vi "HFRR ADV v041.vi"() -> ()   [LabVIEW 2025] (continued)
            n1752 = property on="Port 3" class="Bool (strict)"("Visible"=w2089) -> ()  [unwired: 2 in, 2 out]
          }
        }
        n1753 = Wait (ms)(milliseconds to wait=u32 40) -> ()  [unwired: 1 out]
        n1754 = case shown="True" w2074 {
          tunnel: [w2086 errorcluster {"status"=TRUE, "code"=0, "source"="Init"} ("error out")] -> w2075
          tunnel: w2078 -> [w2086 _]
          frame False {
          }
          frame True {
          }
        }
        n1755 = case shown="Error" w2075 {
          selector: w2075 -> [w2096 w2114]
          tunnel: [w2099 w2118] -> w2085
          tunnel: [w2098 w2112] -> w2084
          tunnel: w2076 -> [w2097 w2116]
          frame No Error {
            n1756 = property class="Instr"(reference=w2097, error in=w2096) -> (reference out=w2094:refnum<visa-resource-name>, error out=w2095:errorcluster, "Serial Settings:Number of Bytes at Serial Port"=w2091:u32)
            n1757 = Greater?(x=w2091, y=u32 5) -> (0:w2090:bool)
            n1758 = Not(x=w2090) -> (.not. x?=→"Port 1a":bool)
            n1759 = while {
              tunnel: [w2107] -> w2098
              tunnel: [w2106] -> w2099
              tunnel: w2095 -> [w2105]
              tunnel: w2094 -> [w2104]
              stop <- TRUE stop-if-true
              n1760 = property class="Instr" props=["Serial Settings:Number of Bytes at Serial Port"](reference=w2104, error in=w2105) -> (reference out=w2109:refnum<visa-resource-name>, error out=w2108:errorcluster)  [unwired: 1 out]
              n1761 = VISA Read(VISA resource name=w2109, byte count=u32 50, error in (no error)=w2108) -> (VISA resource name out=w2106:refnum<visa-resource-name>, read buffer=w2101:string, error out=w2107:errorcluster)  [unwired: 1 out]
              n1762 = Wait (ms)(milliseconds to wait=u32 5) -> ()  [unwired: 1 out]
            }
          }
          frame Error {
            w2124 = u16 0 items=["None", "XON/XOFF", "RTS/CTS", "XON/XOFF & RTS/CTS", "DTR/DSR", "XON/XOFF & DTR/DSR"] ("flow control (0:none)  2")
            w2122 = u16 10 items=["1.0"=10, "1.5"=15, "2.0"=20] ("stop bits 2")
            w2120 = u16 0 items=["None", "Odd", "Even", "Mark", "Space"] ("parity 2")
            w2121 = u32 10000  # timeout (10sec)
            n1763 = VISA Close(VISA resource name=w2116, error in (no error)=w2114) -> (error out=w2117:errorcluster)
            n1764 = local write "Port 1a"(FALSE ("Port 1a")) -> ()
            n1765 = local read "Com Port 1"() -> (w2111:refnum<visa-resource-name>)
            n1766 = call <vilib>:"Clear Errors.vi"("error in (no error)"=w2117) -> ("error out"=w2115:errorcluster)  [unwired: 5 in, 1 out]
            n1767 = call-poly "VISA Configure Serial Port"("VISA resource name"=w2111, "timeout (10sec)"=w2121, "baud rate (9600)"=u32 250000 ("baud rate  2"), "data bits (8)"=u16 8 ("data bits  2"), "parity (0:none)"=w2120, "error in (no error)"=w2115, "stop bits (10: 1 bit)"=w2122, "flow control (0:none)"=w2124) -> ("VISA resource name out"=w2125:refnum<visa-resource-name>, "error out"=w2126:errorcluster)  [unwired: 6 in]
            n1768 = flat-sequence {
              tunnel: w2125 -> [w2128]
              tunnel: w2126 -> [w2127]
              tunnel: [w2128] -> w2118
              tunnel: [w2127] -> w2112
              frame #0 {
                n1769 = Wait (ms)(milliseconds to wait=u32 50) -> ()  [unwired: 1 out]
              }
            }
            "Residual Uno" <- ""
          }
        }
        n1770 = local read "Quit"() -> (w2073:bool)
        "Error Uno" <- w2078
      }
      n1771 = VISA Close(VISA resource name=w2071, error in (no error)=w2070) -> (error out=w2068:errorcluster)
      n1772 = call <vilib>:"Clear Errors.vi"("error in (no error)"=w2068) -> ()  [unwired: 5 in, 2 out]
    }
    frame Enabled {
    }
  }
  n1773 = while {
    stop <- w2139 stop-if-true
    # "V0OLTAGE TO STROKE (peice vise calibration)"
    n1774 = local read "LVDT MIN"() -> (w2131:dbl)
    n1775 = local read "LVDT Peak"() -> (w2130:dbl)
    n1776 = Wait (ms)(milliseconds to wait=u32 10) -> ()  [unwired: 1 out]
    n1777 = formula code="// Dynamic Parameterized Linear Interpolation Node\n// Inputs: vpp_val, voltages (Array), distances (Array)\n// Outputs: stroke\n\nint i = 0;\nint segments = 11; // 12 points make 11 interpolation segments\n\n// 1. Lower Boundary Clamp\nif (vpp_val <= voltages[0]) {\n    stroke = distances[0];\n}\n// 2. Upper Boundary Clamp\nelse if (vpp_val >= voltages[segments]) {\n    stroke = distances[segments];\n}\n// 3. Dynamic Segment Search Loop\nelse {\n    stroke = distances[0]; // Fallback baseline\n    for (i = 0; i < segments; i++) {\n        if (vpp_val >= voltages[i] && vpp_val <= voltages[i+1]) {\n            // Standard linear interpolation formula using array lookups\n            stroke = distances[i] + (vpp_val - voltages[i]) * (distances[i+1] - distances[i]) / (voltages[i+1] - voltages[i]);\n            break; // Segment found, safely exit the loop\n        }\n    }\n}"("vpp_val"=w2130, "voltages"="calibration values", "distances"="STROKE") -> ("stroke"=→"LVDT STROKE":dbl)
    n1778 = local read "Calibration Tare Value"() -> (w2135:dbl)
    n1779 = local read "Calibration Tare"() -> (w2133:bool)
    n1780 = Subtract(x=w2131, y=w2135) -> (x-y=→"LVDT STROKE  Calibration":dbl)
    n1781 = case shown="True" w2133 {
      selector: w2133 -> [_ w2141]
      tunnel: w2131 -> [_ w2142]
      frame False {
      }
      frame True {
        n1782 = Not(x=w2141) -> (.not. x?=w2140:bool)
        n1783 = local write "Calibration Tare"(w2140) -> ()
        "Calibration Tare Value" <- w2142
      }
    }
    n1784 = local read "Quit"() -> (w2139:bool)
  }
  n1785 = while {
    stop <- w2165 stop-if-true
    n1786 = local read "Due read"() -> (w2163:string)
    n1787 = call <vilib>:"High Resolution Polling Wait.vi"("seconds to wait"=0.02) -> ()  [unwired: 10 in, 1 out]
    n1788 = local read "Frictioin Force Raw"() -> (w2145:dbl)
    n1789 = Spreadsheet String To Array(delimiter (Tab)=";", format string="", spreadsheet string=w2163, array type (2D Dbl)=string[] []) -> (array=w2160:string[])
    n1790 = Fract/Exp String To Number(string=w2160) -> (number=w2159:dbl[])  [unwired: 3 in, 1 out]
    n1791 = call <vilib>:"Median Filter PtByPt.vi"("rank"=2, "x"=w2145) -> ("Filtered x"=→"Friction":dbl)  [unwired: 2 in, 1 out]
    n1792 = Index Array(array=w2159) -> (element #1=→"Sample Temperature":dbl, element #2=→"Target Sample Temperature":dbl, element #3=→"Current Duty Cycle":dbl, element #4=→"Ambient Temperature":dbl, element #5=→"Dac Status":dbl, element #6=→"Vpp":dbl, element #7=→"Active Error Code":dbl, element #8=→"Kp":dbl, element #9=→"Ki":dbl, element #10=→"Kd":dbl, element #11=→"SampleRaw":dbl, element #12=→"AmbRaw":dbl)  [unwired: 12 in]
    n1793 = local read "Quit"() -> (w2165:bool)
  }
  n1794 = while {
    shift-right: [w2179] -> w43
    shift-left: _ -> [w2171]
    shift-right: [w2166] -> w42
    shift-left: errorcluster {"status"=FALSE, "code"=0, "source"="Init"} ("error out") -> [w2173]
    tunnel: [w2168] -> w46
    tunnel: [w2178] -> _
    i -> [w2178]
    stop <- w2168 stop-if-true
    n1795 = local read "Com Port 2"() -> (w2172:refnum<visa-resource-name>)
    n1796 = local read "Port 2a"() -> (w2174:bool)
    n1797 = Unbundle(w2173) -> ("status"=→"Port 4":bool)  [unwired: 2 out]
    n1798 = call <vilib>:"High Resolution Polling Wait.vi"("seconds to wait"=0.02) -> ()  [unwired: 10 in, 1 out]
    n1799 = local read "Port 4"() -> (w2175:bool)
    n1800 = Not Equal?(x=w2172, y=w2171) -> (x != y?=w2170:bool)
    n1801 = Or(x=w2175, y=w2174) -> (x .or. y?=w2177:bool)
    n1802 = case shown="False" w2177 {
      frame False {
        w2182 = TRUE ("Visible")
        n1803 = property on="Port 2a" class="Bool (strict)"("Visible"=w2182) -> ()  [unwired: 2 in, 2 out]
        n1804 = property on="Port 4" class="Bool (strict)"("Visible"=w2182) -> ()  [unwired: 2 in, 2 out]
      }
      frame True {
        w2183 = TRUE ("Visible")
        n1805 = property on="Port 2a" class="Bool (strict)"("Visible"=w2183) -> ()  [unwired: 2 in, 2 out]
        n1806 = property on="Port 4" class="Bool (strict)"("Visible"=w2183) -> ()  [unwired: 2 in, 2 out]
      }
    }
    n1807 = case shown="True" w2170 {
      tunnel: [w2180 errorcluster {"status"=TRUE, "code"=0, "source"="Init"} ("error out")] -> w2169
      tunnel: w2173 -> [w2180 _]
      frame False {
      }
      frame True {
      }
    }
    n1808 = case shown="No Error" w2169 {
      selector: w2169 -> [w2196 w2227]
      tunnel: [w2189 w2232] -> w2179
      tunnel: [w2197 w2225] -> w2166
      tunnel: w2171 -> [w2198 w2230]
      frame No Error {
        n1809 = property class="Instr" props=["Serial Settings:Number of Bytes at Serial Port"](reference=w2198, error in=w2196) -> (reference out=w2190:refnum<visa-resource-name>, error out=w2195:errorcluster)  [unwired: 1 out]
        n1810 = while {
          tunnel: [w2206] -> w2191
          tunnel: [w2205] -> w2192
          tunnel: w2195 -> [w2204]
          tunnel: w2190 -> [w2203]
          tunnel: [w2202] -> _
          i -> [w2202]
          stop <- TRUE stop-if-true
          n1811 = property class="Instr" props=["Serial Settings:Number of Bytes at Serial Port"](reference=w2203, error in=w2204) -> (reference out=w2208:refnum<visa-resource-name>, error out=w2207:errorcluster)  [unwired: 1 out]
          n1812 = VISA Read(VISA resource name=w2208, byte count=u32 1000, error in (no error)=w2207) -> (VISA resource name out=w2205:refnum<visa-resource-name>, read buffer=→"Due read":string, error out=w2206:errorcluster)  [unwired: 1 out]
        }
        n1813 = local read "Due Write"() -> (w2188:string)
        n1814 = call <vilib>:"Trim Whitespace.vi"("string"=w2188) -> ("trimmed string"=w2187:string)  [unwired: 1 in]
        n1815 = Not Equal?(x=w2187, y="") -> (x != y?=w2193:bool)
        n1816 = VISA Flush I/O Buffer(VISA resource name=w2192) -> (VISA resource name out=w2185:refnum<visa-resource-name>, error out=→"error out 10":errorcluster)  [unwired: 2 in]
        n1817 = case shown="True" w2193 {
          tunnel: w2185 -> [w2210 w2215]
          tunnel: [w2210 w2219] -> w2189
          tunnel: w2191 -> [w2209 w2214]
          tunnel: [w2209 w2217] -> w2197
          tunnel: w2187 -> [_ w2213]
          tunnel: [_ w2216] -> _
          frame False {
            # "DATA  WRITE LOOP"
          }
          frame True {
            n1818 = Concatenate Strings(w2213, "\r\n") -> (w2212:string)
            n1819 = VISA Write(VISA resource name=w2215, write buffer=w2212, error in (no error)=w2214) -> (VISA resource name out=w2219:refnum<visa-resource-name>, return count=w2216:u32, error out=w2218:errorcluster)
            n1820 = flat-sequence {
              tunnel: w2218 -> [w2221]
              tunnel: [w2221] -> w2217
              frame #0 {
                n1821 = local write "Due Write"("" ("Command")) -> ()
                n1822 = Wait (ms)(milliseconds to wait=u32 5) -> ()  [unwired: 1 out]
              }
            }
          }
        }
        "Port 2a" <- TRUE ("Port 2a")
      }
      frame Error {
        w2238 = u16 0 items=["None", "XON/XOFF", "RTS/CTS", "XON/XOFF & RTS/CTS", "DTR/DSR", "XON/XOFF & DTR/DSR"] ("flow control (0:none)  2")
        w2236 = u16 10 items=["1.0"=10, "1.5"=15, "2.0"=20] ("stop bits 2")
        w2234 = u16 0 items=["None", "Odd", "Even", "Mark", "Space"] ("parity 2")
        w2235 = u32 10000  # timeout (10sec)
        n1823 = VISA Clear(VISA resource name=w2230, error in (no error)=w2227) -> (VISA resource name out=w2229:refnum<visa-resource-name>, error out=w2228:errorcluster)
        n1824 = VISA Close(VISA resource name=w2229, error in (no error)=w2228) -> (error out=w2231:errorcluster)
        n1825 = call <vilib>:"Clear Errors.vi"("error in (no error)"=w2231) -> ()  [unwired: 5 in, 2 out]
        n1826 = local write "Port 2a"(FALSE ("Port 2a")) -> ()
        n1827 = local read "Com Port 2"() -> (w2224:refnum<visa-resource-name>)
        "visa due" <- w2224
        n1828 = call-poly "VISA Configure Serial Port"("VISA resource name"=w2224, "timeout (10sec)"=w2235, "baud rate (9600)"=u32 250000 ("baud rate  2"), "data bits (8)"=u16 8 ("data bits  2"), "parity (0:none)"=w2234, "stop bits (10: 1 bit)"=w2236, "flow control (0:none)"=w2238) -> ("VISA resource name out"=w2239:refnum<visa-resource-name>, "error out"=w2240:errorcluster)  [unwired: 7 in]
        n1829 = flat-sequence {
          tunnel: w2239 -> [w2242]
          tunnel: w2240 -> [w2241]
          tunnel: [w2242] -> w2232
          tunnel: [w2241] -> w2225
          frame #0 {
            n1830 = Wait (ms)(milliseconds to wait=u32 50) -> ()  [unwired: 1 out]
          }
        }
        "Residual Due" <- ""
      }
    }
    "error out 9" <- w2166
    n1831 = local read "Quit"() -> (w2168:bool)
    "Error Due" <- w2173
  }
  n1832 = local write "FRICVALZ"(0.0 ("FRICVALZ")) -> ()
  n1833 = property on="RUN" class="Bool (strict)"("Visible"=TRUE) -> ()  [unwired: 2 in, 2 out]
  n1834 = while {
    tunnel: [w2257] -> _
    tunnel: [w2244] -> w56
    i -> [w2257]
    stop <- w2244 stop-if-true
    n1835 = local read "conststatus"() -> (w2248:dbl)
    n1836 = local read "Main Tab"() -> (w2246:T2)
    n1837 = local read "EDIT"() -> (w2263:bool)
    n1838 = local read "Rate"() -> (w2262:dbl)
    n1839 = case shown="True" w2263 {
      tunnel: [FALSE TRUE] -> _
      frame False {
      }
      frame True {
      }
    }
    n1840 = Equal?(x=w2246, y=T29."About" ("Main Tab")) -> (x = y?=w2255:bool)
    n1841 = Equal?(x=w2248, y=0.0) -> (x = y?=w2249:bool)
    n1842 = Divide(x=1.0, y=w2262) -> (x/y=w2258:dbl)
    "Time 2" <- w2258
    n1843 = case shown="True" w2249 {
      frame False {
      }
      frame True {
        # "C:\\WinDucom\\calibrate WO 2391.dcf"
        n1844 = local write "Lan flag"(22) -> ()
        n1845 = local write "conststatus"(10.0 ("rpm value : 2")) -> ()
        n1846 = String To Path(string="C:\\LAB-IQ\\calibrate WO 2465.dcf") -> (path=w2269:path)
        n1847 = Open/Create/Replace File "Open File"(file path (use dialog)=w2269) -> (refnum out=w2267:refnum<file>)  [unwired: 5 in, 2 out]
        n1848 = for {
          N: 23 -> [_]
          tunnel: w2267 -> [w2278]
          i -> [w2272]
          (unwired) TRUE ("line mode (F)")
          n1849 = Read from Text File "Read File"(file (use dialog)=w2278) -> (text=w2277:string)  [unwired: 3 in, 3 out]
          n1850 = Match Pattern(string=w2277, regular expression="]") -> (after substring=w2275:string)  [unwired: 1 in, 3 out]
          n1851 = String Subset(string=w2277, offset (0)=5, length (rest)=10 ("length (rest)")) -> (substring=w2270:string)
          n1852 = Fract/Exp String To Number(string=w2270) -> (number=w2271:dbl)  [unwired: 3 in, 1 out]
          n1853 = Match Pattern(string=w2275, regular expression="-") -> (before substring=w2273:string)  [unwired: 1 in, 3 out]
          n1854 = case shown="10" w2272 {
            tunnel: w2271 -> [_ _ _ _ _ _ _ _ _ _ w2285 _ _ _ _ _ _ _ _ _ _ _ _ _]
            tunnel: w2273 -> [_ _ _ _ w2281 w2282 w2283 _ _ _ _ _ _ _ _ _ _ _ _ _ w2286 w2287 w2288 _]
            frame 0 {
            }
            frame 1 {
            }
            frame 2 {
            }
            frame 3 {
            }
            frame 4 {
              n1855 = local write "Com Port 1"(w2281) -> ()
            }
            frame 5 {
              n1856 = local write "Com Port 2"(w2282) -> ()
              n1857 = local write "visa due"(w2282) -> ()
            }
            frame 6 {
              n1858 = String To Path(string=w2283) -> (path=w2284:path)
              n1859 = local write "File Path"(w2284) -> ()
              "String" <- w2283
            }
            frame 7 {
            }
            frame 8 {
            }
            frame 9 {
            }
            frame 10 {
              n1860 = local write "Language Selection"(w2285) -> ()
            }
            frame 11 {
            }
            frame 12 {
            }
            frame 13 {
            }
            frame 14 {
            }
            frame 15 {
            }
            frame 16 {
            }
            frame 17 {
            }
            frame 18 {
            }
            frame 21 {
            }
            frame 22 {
              n1861 = local write "Com Port 3"(w2286) -> ()
            }
            frame 20 {
              n1862 = local write "Camera Port :"(w2287) -> ()
            }
            frame 19 {
              n1863 = local write "C3 :"(w2288) -> ()
            }
            frame 23, Default {
            }
          }
        }
      }
    }
    n1864 = Select(t=u32 2500 ("milliseconds to wait"), s=w2255, f=u32 500 ("milliseconds to wait")) -> (s? t:f=w2253:u32)
    n1865 = Multiply(x=w2258, y=w2253) -> (x*y=w2260:dbl)
    n1866 = call "Elapsed Time2"("Time Target (s)"=w2260, "Auto Reset"=TRUE) -> ("Time has Elapsed"=w2250:bool)  [unwired: 10 in, 7 out]
    n1867 = case shown="True" w2250 {
      frame False {
      }
      frame True {
        n1868 = stacked-sequence {
          frame #0 {
            # "DATA PROCESSING"
            # "115 mV/N"
            n1869 = local read "Sample Temperature"() -> (w2291:dbl)
            n1870 = local read "RH Numeric:"() -> (→"Humidity ( %RH )":dbl)
            n1871 = local read "FRICVALZ"() -> (w2308:dbl)
            n1872 = local read "Friction"() -> (w2294:dbl)
            n1873 = call <vilib>:"Mean PtByPt.vi"("x"=w2291, "sample length"=100) -> ("mean"=w2290:dbl)  [unwired: 2 in, 1 out]
            "TEMP 2" <- w2290
            "TEMP 3" <- w2290
            n1874 = Subtract(x=w2294, y=w2308) -> (x-y=w2303:dbl)
            "FF 2" <- w2303
            "FF 4" <- w2303
            n1875 = local read "Ambient Temperature"() -> (→"AIR TEMP":dbl)
            n1876 = local read "TEMP"() -> (w2307:dbl)
            n1877 = local write "FF 3"(w2303) -> ()
            n1878 = Compound Arithmetic op=OR("FRICVALZ 4", "FRICVALZ 3", "FRICVALZ 2") -> (w2299:bool)
            n1879 = case shown="True" w2299 {
              tunnel: w2294 -> [_ w2314]
              frame False {
              }
              frame True {
                w2313 = FALSE ("FRICVALZ")
                n1880 = local write "FRICVALZ 3"(w2313) -> ()
                n1881 = local write "FRICVALZ 2"(w2313) -> ()
                n1882 = local write "FRICVALZ 4"(w2313) -> ()
                "FRICVALZ" <- w2314
              }
            }
            n1883 = Not A Number/Path/Refnum?(number/path/refnum=w2307) -> (NaN/Path/Refnum?=w2306:bool)
            n1884 = Not A Number/Path/Refnum?(number/path/refnum=w2303) -> (NaN/Path/Refnum?=w2305:bool)
            n1885 = Divide(x=w2303, y=1.96) -> (x/y=w2300:dbl)
            n1886 = Compound Arithmetic op=OR(w2306, w2305) -> (w2304:bool)
            n1887 = Not A Number/Path/Refnum?(number/path/refnum=w2300) -> (NaN/Path/Refnum?=w2301:bool)
            n1888 = case shown="True" w2304 {
              frame False {
              }
              frame True {
                n1889 = local write "TEMP"(0.0 ("TEMP")) -> ()
                n1890 = local write "FF 2"(0.0 ("FF 2")) -> ()
                n1891 = local write "reinit"(TRUE ("reinit")) -> ()
              }
            }
            n1892 = local write "TEMP"(w2290) -> ()
            n1893 = Select(t=0.0, s=w2301, f=w2300) -> (s? t:f=w2293:dbl)
            "COF 2" <- w2293
            n1894 = local write "COF 3"(w2293) -> ()
          }
        }
      }
    }
    n1895 = Wait (ms)(milliseconds to wait=u32 50) -> ()  [unwired: 1 out]
    n1896 = local read "Quit"() -> (w2244:bool)
    "Rate" <- 2500.0 ("No of Samples")
  }
  n1897 = while {
    tunnel: [w2334] -> _
    tunnel: [w2317] -> w58
    tunnel: w3 -> [_]
    i -> [w2334]
    stop <- w2317 stop-if-true
    # "C:\\LAB-IQ-NXT\\Scar View.exe"
    n1898 = local read "OK Button 16"() -> (w2324:bool)
    n1899 = local read "Main Tab"() -> (w2318:T2)
    n1900 = local read "service 3"() -> (w2319:bool)
    n1901 = local read "OPEN 6"() -> (w2321:bool)
    n1902 = local read "EDIT 2"() -> (w2323:bool)
    n1903 = flat-sequence {
      frame #0 {
        n1904 = stacked-sequence {
          frame #0 {
            n1905 = local read "EDIT"() -> (w2812:bool)
            n1906 = case shown="False" w2812 {
              tunnel: [u8 2 ("Disabled") u8 0 ("Disabled")] -> _
              frame False {
                w2814 = FALSE
                n1907 = local write "Password"("") -> ()
                n1908 = local write "x = y?"(w2814) -> ()
                n1909 = property on="Password" class="Str"("Visible"=w2814) -> ()  [unwired: 2 in, 2 out]
              }
              frame True {
                n1910 = property on="Password" class="Str"("Visible"=TRUE) -> ()  [unwired: 2 in, 2 out]
              }
            }
            "dipl pwd" <- "@143$\n" ("dipl pwd")
          }
          frame #1 {
          }
          frame #2 {
          }
          frame #3 {
          }
          frame #4 {
            n1911 = String To Byte Array(string="Password") -> (unsigned byte array=w2825:u8[])
            n1912 = Search 1D Array(1D array=w2825, element=u8 10) -> (index of element=w2823:i32)  [unwired: 1 in]
            n1913 = Index Array(array=w2825, index=w2823) -> (element=w2824:u8)
            n1914 = Equal?(x=w2824, y=10) -> (x = y?=w2820:bool)
            n1915 = case shown="True" w2820 {
              frame False {
              }
              frame True {
                # "password"
                # "password"
                n1916 = local read "Password"() -> (w2837:string)
                n1917 = String To Byte Array(string=w2837) -> (unsigned byte array=w2840:u8[])
                n1918 = String To Byte Array(string="@143$\n") -> (unsigned byte array=w2827:u8[])
                n1919 = Array Size(array=w2840) -> (size(s)=w2836:i32)
                n1920 = Array Size(array=w2827) -> (size(s)=w2832:i32)
                n1921 = for {
                  N: w2836 -> [_]
                  tunnel: w2840 -> [w2853]
                  tunnel: [w2851] -> w2841 mode=indexing
                  tunnel: w2836 -> [w2848]
                  i -> [w2849]
                  n1922 = Decrement(x=w2848) -> (x-1=w2847:i32)
                  n1923 = Index Array(array=w2853, index=w2849) -> (element=w2852:u8)
                  n1924 = Equal?(x=w2849, y=w2847) -> (x = y?=w2846:bool)
                  n1925 = Number To Decimal String(number=w2852) -> (decimal integer string=w2850:string)  [unwired: 1 in]
                  n1926 = Select(t="", s=w2846, f="\r") -> (s? t:f=w2843:string)
                  n1927 = Concatenate Strings(w2850, w2843) -> (w2851:string)
                }
                n1928 = for {
                  N: w2832 -> [_]
                  tunnel: w2827 -> [w2864]
                  tunnel: [w2862] -> w2830 mode=indexing
                  tunnel: w2832 -> [w2859]
                  i -> [w2860]
                  n1929 = Decrement(x=w2859) -> (x-1=w2858:i32)
                  n1930 = Index Array(array=w2864, index=w2860) -> (element=w2863:u8)
                  n1931 = Equal?(x=w2860, y=w2858) -> (x = y?=w2857:bool)
                  n1932 = Number To Decimal String(number=w2863) -> (decimal integer string=w2861:string)  [unwired: 1 in]
                  n1933 = Select(t="", s=w2857, f="\r") -> (s? t:f=w2854:string)
                  n1934 = Concatenate Strings(w2861, w2854) -> (w2862:string)
                }
                n1935 = local read "file path"() -> (w2826:path)
                n1936 = call <vilib>:"Read Characters From File.vi"("file path (dialog if empty)"=w2826) -> ("character string"=w2839:string)  [unwired: 5 in, 3 out]
                "string" <- w2839
                n1937 = flat-sequence {
                  tunnel: [w2842] -> _
                  frame #0 {
                    w2842 = ""
                    n1938 = local write "Password"(w2842) -> ()
                  }
                }
                n1939 = Concatenate Strings(w2830) -> (w2831:string)
                n1940 = Concatenate Strings(w2839) -> (w2838:string)
                n1941 = Concatenate Strings(w2841) -> (w2834:string)
                n1942 = Equal?(x=w2834, y=w2838) -> (x = y?=w2829:bool)
                n1943 = Equal?(x=w2834, y=w2831) -> (x = y?=w2835:bool)
                n1944 = Or(x=w2829, y=w2835) -> (x .or. y?=→"x = y?":bool)
              }
            }
          }
        }
        n1945 = local read "x = y?"() -> (w2810:bool)
        n1946 = And(x="EDIT", y=w2810) -> (x .and. y?=w2808:bool)
        n1947 = case shown="True" w2808 {
          tunnel: [u8 2 ("Disabled") u8 0 ("Disabled")] -> w2807
          tunnel: [w3014 TRUE ("Visible")] -> w2806
          frame False {
            w3014 = FALSE ("Visible")
            n1948 = local write "EDIT 2"(w3014) -> ()
          }
          frame True {
          }
        }
        n1949 = case shown="True" "SAVE" {
          frame False {
          }
          frame True {
            n1950 = stacked-sequence {
              seq-local: [w2869 _ _] -> [_ w3010 _]
              frame #0 {
                w2865 = 0.0 ("number")
                w2866 = 0.0 ("number")
                (unwired) i16 5 ("precision (6)")
                # "[CH1]    - FF\n[CH2]   - TEMPERATURE\n[CH3]    - Humidity\n[CH4]    - AIR TEMP\n[CH5]\\- Visa Uno\n[CH6] \\- Visa Due\n[CH7]  \\- file path\n[CH8]   - Displacement Gain\n[CHA]   - Stroke Gain\n[CHB]   - Stroke PID Gain\n[CHC]   -Language Selection\n[CHD]   -Power +\n[CHE]   -Power_\n[CHF]   -Heater\n[CHG]   -Humidity Wet\n[CHH]   -Humidity Dry\n[CHI]   -Integral Time"
                n1951 = local read "Language Selection"() -> (w2912:enum16{"English", "Russian"})
                n1952 = Path To String(path="File Path") -> (string=w2928:string)
                n1953 = Number To Fractional String(number=w2865, width (-)=i16 10 ("precision (6)"), precision (6)=i16 5) -> (F-format string=w2919:string)  [unwired: 1 in]
                n1954 = Number To Fractional String(number=w2912, width (-)=i16 10 ("precision (6)"), precision (6)=i16 5) -> (F-format string=w2908:string)  [unwired: 1 in]
                n1955 = Number To Fractional String(number=w2866, width (-)=i16 10 ("precision (6)"), precision (6)=i16 5) -> (F-format string=w2902:string)  [unwired: 1 in]
                n1956 = Number To Fractional String(number=w2866, width (-)=i16 10 ("precision (6)"), precision (6)=i16 5) -> (F-format string=w2899:string)  [unwired: 1 in]
                n1957 = Number To Fractional String(number=w2866, width (-)=i16 10 ("precision (6)"), precision (6)=i16 5) -> (F-format string=w2894:string)  [unwired: 1 in]
                n1958 = Number To Fractional String(number=w2866, width (-)=i16 10 ("precision (6)"), precision (6)=i16 5) -> (F-format string=w2891:string)  [unwired: 1 in]
                n1959 = Number To Fractional String(number=w2866, width (-)=i16 10 ("precision (6)"), precision (6)=i16 5) -> (F-format string=w2886:string)  [unwired: 1 in]
                n1960 = local read "Com Port 1"() -> (w2868:refnum<visa-resource-name>)
                n1961 = local read "Com Port 2"() -> (w2867:refnum<visa-resource-name>)
                n1962 = Concatenate Strings(w2928, "\\" ("string")) -> (w2927:string)
                n1963 = Number To Fractional String(number=w2865, width (-)=i16 10 ("precision (6)"), precision (6)=i16 5) -> (F-format string=w2960:string)  [unwired: 1 in]
                n1964 = Number To Fractional String(number=w2865, width (-)=i16 10 ("precision (6)"), precision (6)=i16 5) -> (F-format string=w2959:string)  [unwired: 1 in]
                n1965 = Number To Fractional String(number=w2865, width (-)=i16 10 ("precision (6)"), precision (6)=i16 5) -> (F-format string=w2953:string)  [unwired: 1 in]
                n1966 = Number To Fractional String(number=w2865, width (-)=i16 10 ("precision (6)"), precision (6)=i16 5) -> (F-format string=w2947:string)  [unwired: 1 in]
                n1967 = Number To Fractional String(number=w2865, width (-)=i16 10 ("precision (6)"), precision (6)=i16 5) -> (F-format string=w2920:string)  [unwired: 1 in]
                n1968 = Concatenate Strings("[CHA]" ("string"), w2919, "- Stroke Gain" ("string"), "\r") -> (w2913:string)
                n1969 = Concatenate Strings("[CHC]" ("string"), w2908, "-Language Selection" ("string"), "\r") -> (w2905:string)
                n1970 = Concatenate Strings("[CHD]" ("string"), w2902, "-Power +" ("string"), "\r") -> (w2884:string)
                n1971 = Concatenate Strings("[CHG]" ("string"), w2891, "-Humidity Wet" ("string"), "\r") -> (w2881:string)
                n1972 = Concatenate Strings("[CHH]" ("string"), w2886, "-Humidity Dry" ("string"), "\r") -> (w2880:string)
                n1973 = Concatenate Strings("[CH1]" ("string"), w2960, " - FF" ("string"), "\r") -> (w2958:string)
                n1974 = Concatenate Strings("[CH2]" ("string"), w2959, " - TEMPERATURE" ("string"), "\r") -> (w2957:string)
                n1975 = Concatenate Strings("[CH3]" ("string"), w2953, " - Humidity" ("string"), "\r") -> (w2950:string)
                n1976 = Concatenate Strings("[CH4]" ("string"), w2947, " - AIR TEMP" ("string"), "\r") -> (w2943:string)
                n1977 = Concatenate Strings("[CH5]" ("string"), w2868, "- Visa Uno" ("string"), "\r") -> (w2936:string)
                n1978 = Concatenate Strings("[CH6]" ("string"), w2867, "- Visa Due" ("string"), "\r") -> (w2931:string)
                n1979 = Concatenate Strings("[CH7]" ("string"), w2927, "- file path" ("string"), "\r") -> (w2930:string)
                n1980 = Concatenate Strings("[CH8]" ("string"), w2920, "- Displacement Gain" ("string"), "\r") -> (w2923:string)
                n1981 = Concatenate Strings("[CHE]" ("string"), w2899, "-Power_" ("string"), "\r") -> (w2883:string)
                n1982 = Concatenate Strings("[CHF]" ("string"), w2894, "-Heater" ("string"), "\r") -> (w2882:string)
                n1983 = Concatenate Strings(w2958, w2957, w2950, w2943, w2936, w2931, w2930, w2923, w2913, w2905, w2884, w2883, w2882, w2881, w2880) -> (w2869:string)
                "gain" <- w2869
              }
              frame #1 {
                w2971 = 0.0 ("number")
                n1984 = local read "Camera Port :"() -> (w2974:string)
                n1985 = local read "C3 :"() -> (w2982:refnum<visa-resource-name>)
                n1986 = local read "Com Port 3"() -> (w2983:refnum<visa-resource-name>)
                n1987 = Concatenate Strings("[CH8]" ("string"), w2974, "- Visa Camera" ("string"), "\r") -> (w2973:string)
                n1988 = Concatenate Strings("[CH7]" ("string"), w2982, "- Visa Humidity" ("string"), "\r") -> (w2978:string)
                n1989 = Number To Fractional String(number=w2971, width (-)=i16 10 ("precision (6)"), precision (6)=i16 5) -> (F-format string=w2998:string)  [unwired: 1 in]
                n1990 = Concatenate Strings("[CHL]" ("string"), w2983, "- Visa humid" ("string"), "\r") -> (w2986:string)
                n1991 = Number To Fractional String(number=w2971, width (-)=i16 10 ("precision (6)"), precision (6)=i16 5) -> (F-format string=w3005:string)  [unwired: 1 in]
                n1992 = Concatenate Strings("[CHK]" ("string"), w2998, "-TEMP INTERCEPT" ("string"), "\r") -> (w2994:string)
                n1993 = Concatenate Strings("[SNO]" ("string"), "" ("string"), "-" ("string"), "\r") -> (w2991:string)
                n1994 = Concatenate Strings("[CHJ]" ("string"), w3005, "-AIR TEMP INTERCEPT" ("string"), "\r") -> (w2995:string)
                n1995 = String To Path(string="C:\\LAB-IQ\\calibrate WO 2465.dcf") -> (path=w2984:path)
                n1996 = Concatenate Strings(w3010, w2995, w2994, w2991, w2986, w2978, w2973) -> (w3009:string)
                n1997 = call <vilib>:"Write Characters To File.vi"("append to file? (new file:F)"=FALSE, "character string"=w3009, "file path (dialog if empty)"=w2984) -> ()  [unwired: 2 in, 1 out]
              }
              frame #2 {
                n1998 = local write "Lan flag"(0.0 ("Lan flag")) -> ()
                n1999 = local write "conststatus"(0.0 ("rpm value : 2")) -> ()
                n2000 = local write "SAVE"(FALSE ("OK Button 14")) -> ()
              }
            }
          }
        }
        n2001 = property on="EDIT 2" class="Bool (strict)"("Visible"=w2806) -> ()  [unwired: 2 in, 2 out]
        n2002 = property on="SAVE" class="Bool (strict)"("Visible"=w2806) -> ()  [unwired: 2 in, 2 out]
        n2003 = property on="visa due" class="CmbBox"("Disabled"=w2807) -> ()  [unwired: 2 in, 2 out]
        n2004 = property on="File Path" class="Path"("Disabled"=w2807) -> ()  [unwired: 2 in, 2 out]
        n2005 = property on="Language Selection" class="Enum (strict)"("Visible"=w2806) -> ()  [unwired: 2 in, 2 out]
        n2006 = property on="SPEED OUT:" class="DigNum (strict)"("Disabled"=w2807) -> ()  [unwired: 2 in, 2 out]
      }
    }
    n2007 = local read "RUN"() -> (w2333:bool)
    n2008 = local read "RUN"() -> (w2331:bool)
    n2009 = case shown="True" "EDIT 3" {
      frame False {
      }
      frame True {
        n2010 = local write "EDIT 3"(FALSE ("EDIT 3")) -> ()
        n2011 = local write "Main Tab"(T2."About" ("Main Tab")) -> ()
      }
    }
    n2012 = case shown="False" w2333 {
      frame False {
        n2013 = local read "stopT"() -> (w3021:bool)
        n2014 = case shown="True" w3021 {
          frame False {
          }
          frame True {
            n2015 = local write "stopT"(FALSE) -> ()
          }
        }
      }
      frame True {
        "stopT" <- TRUE
      }
    }
    n2016 = case shown="False" w2331 {
      frame False {
      }
      frame True {
      }
    }
    n2017 = case shown="True" w2323 {
      frame False {
        n2018 = property on="Password 2" class="Str"("Visible"=FALSE) -> ()  [unwired: 2 in, 2 out]
        n2019 = local write "Password 2"("" ("Password")) -> ()
      }
      frame True {
        n2020 = property on="Password 2" class="Str"("Visible"=TRUE) -> ()  [unwired: 2 in, 2 out]
        n2021 = Equal?(x="Password 2", y="HFRR1234") -> (x = y?=w2346:bool)
        n2022 = case shown="True" w2346 {
          tunnel: "Password 2" -> [w2349 _]
          frame False {
            n2023 = String Length(string=w2349) -> (length=w2350:i32)
            n2024 = Greater Than 0?(x=w2350) -> (x > 0?=w2348:bool)
            n2025 = case shown="False" w2348 {
              frame False {
                n2026 = property on="Password 2" class="Str"("Caption.Text"="Password (Advance Setting)") -> ()  [unwired: 2 in, 2 out]
              }
              frame True {
                n2027 = property on="Password 2" class="Str"("Caption.Text"="Incorrect Password!") -> ()  [unwired: 2 in, 2 out]
              }
            }
          }
          frame True {
            n2028 = local write "EDIT 2"(FALSE ("EDIT 2")) -> ()
            n2029 = local write "Password 2"("" ("Password")) -> ()
            n2030 = local write "Main Tab"(T2."Advance" ("Main Tab")) -> ()
            n2031 = local write "Main Dashboard Buttons"(T1."Advance" ("Main Dashboard Buttons")) -> ()
          }
        }
      }
    }
    n2032 = case shown="True" "Prog Uno" {
      frame False {
      }
      frame True {
        n2033 = stacked-sequence {
          frame #0 {
            n2034 = Delete(path (use dialog)=path "C:/LAB-IQ-NXT/UNOCOMPILE.bat" ("working directory")) -> ()  [unwired: 4 in, 3 out]
          }
          frame #1 {
            n2035 = local read "Com Port 1"() -> (w2788:refnum<visa-resource-name>)
            n2036 = Concatenate Strings("cmd.exe /c \"mode " ("command line"), w2788, ":1200,n,8,1\"\n" ("command line")) -> (w2793:string)
            n2037 = Concatenate Strings(w2793, "CD\\\nCD WinDucom\navrdude -C avrdude.conf -v -patmega328p -carduino -P" ("command line"), w2788, " -b115200 -D -Uflash:w:UNO_V20.hex:i\n" ("command line"), "\r") -> (w2795:string)
            "STR" <- w2795
            n2038 = call <vilib>:"Write Characters To File.vi"("append to file? (new file:F)"=FALSE, "character string"=w2795, "file path (dialog if empty)"=path "C:/LAB-IQ/UNOCOMPILE.bat" ("working directory")) -> ()  [unwired: 2 in, 1 out]
          }
          frame #2 {
            n2039 = disable-structure shown="Disabled" {
              frame Disabled {
                w2799 = "cmd.exe  /c \"C:\\LAB-IQ-NXT\\UNOCOMPILE.bat\"" ("string")
                n2040 = local write "Prog Uno"(FALSE ("run minimized? (F)")) -> ()
                n2041 = call <vilib>:"System Exec.vi"("expected output size  (4096)"=u32 65535, "run minimized? (F)"=FALSE, "wait until completion? (T)"=TRUE ("run minimized? (F)"), "working directory"=path "C:/LAB-IQ-NXT", "standard input"=w2799, "command line"=w2799) -> ("error out"=w2798:errorcluster, "standard output"=→"String 42":string)  [unwired: 2 in, 2 out]
                "error out 3" <- w2798
                n2042 = flat-sequence {
                  tunnel: w2798 -> [_]
                  frame #0 {
                  }
                }
              }
              frame Enabled {
              }
            }
          }
        }
      }
    }
    n2043 = case shown="\"ISO 12156\"" "TEST STANDARD" {
      frame "ASTM D6079", Default {
        w2768 = 50.0 ("Hz")
        w2769 = 53.0 ("Set Rh")
        w2771 = 1.0 ("Set Strk")
        w2770 = 60.0 ("Set Temp")
        # "astm hide"
        n2044 = local write "NORMAL LOAD"(200.0 ("NORMAL LOAD")) -> ()
        n2045 = local write "Set Strk"(w2771) -> ()
        n2046 = local write "Set Hz"(w2768) -> ()
        n2047 = local write "Set Temp"(w2770) -> ()
        n2048 = local write "Set Rh"(w2769) -> ()
        n2049 = local write "test time"(75.0 ("test time")) -> ()
        n2050 = local write "Set Stroke:"(w2771) -> ()
        n2051 = local write "Set Humidity:"(w2769) -> ()
        n2052 = local write "Set Frequency:"(w2768) -> ()
        n2053 = local write "Set Temperature:"(w2770) -> ()
        "Test Standard" <- "ASTM D6079" ("Test Standard 2")
      }
      frame "ISO 12156" {
        n2054 = local write "Set Strk"(1.0 ("Set Strk")) -> ()
        n2055 = local write "NORMAL LOAD"(200.0 ("NORMAL LOAD")) -> ()
        n2056 = local write "Set Temp"(60.0 ("Set Temp")) -> ()
        n2057 = local write "test time"(75.0 ("test time")) -> ()
        n2058 = local write "Set Hz"(50.0 ("Hz")) -> ()
        n2059 = local write "Set Rh"(53.0 ("Set Rh")) -> ()
      }
      frame "CEC F-096-A-06" {
        n2060 = local write "Set Strk"(1.0 ("Set Strk")) -> ()
        n2061 = local write "NORMAL LOAD"(200.0 ("NORMAL LOAD")) -> ()
        n2062 = local write "Set Temp"(60.0 ("Set Temp")) -> ()
        n2063 = local write "test time"(75.0 ("test time")) -> ()
        n2064 = local write "Set Hz"(50.0 ("Hz")) -> ()
        n2065 = local write "Set Rh"(53.0 ("Set Rh")) -> ()
      }
      frame "Custom" {
      }
    }
    n2066 = Or(x=w2321, y=w2319) -> (x .or. y?=w2320:bool)
    n2067 = case shown="\"About\"" w2318 {
      tunnel: [T29."Acquire" ("Main Tab") T29."Compare Files" ("Main Tab") T29."About" ("Main Tab")] -> w2329
      frame "Acquire", Default {
      }
      frame "Compare Files" {
      }
      frame "About" {
      }
    }
    n2068 = Or(x=w2324, y="OPEN") -> (x .or. y?=w2325:bool)
    n2069 = case shown="True" w2325 {
      tunnel: w2324 -> [_ w2357]
      frame False {
      }
      frame True {
        n2070 = stacked-sequence {
          tunnel: w2357 -> [_ w2424 _ _]
          frame #0 {
            w2373 = "  " ("String 6")
            n2071 = local write "OPEN"(FALSE ("open")) -> ()
            n2072 = local read "string1 2"() -> (w2361:string)
            n2073 = local read "string1 3"() -> (w2360:string)
            n2074 = local read "string1 4"() -> (w2359:string)
            n2075 = property on="OPEN" class="Bool (strict)"("Visible"=FALSE) -> ()  [unwired: 2 in, 2 out]
            n2076 = local write "String 6"(w2373) -> ()
            n2077 = local write "String 7"(w2373) -> ()
            n2078 = local write "String 8"(w2373) -> ()
            n2079 = local write "String 12"(w2373) -> ()
            n2080 = local read "OK Button 16"() -> (w2358:bool)
            n2081 = String To Path(string=w2361) -> (path=w2369:path)
            n2082 = String To Path(string=w2360) -> (path=w2368:path)
            n2083 = String To Path(string=w2359) -> (path=w2367:path)
            n2084 = case shown="True" w2358 {
              tunnel: [w2374 w2375] -> w2362
              frame False {
                n2085 = local read "string1"() -> (w2374:string)
              }
              frame True {
                n2086 = local read "String Indicator 4"() -> (w2375:string)
              }
            }
            n2087 = Open/Create/Replace File "Open File"(file path (use dialog)=w2369) -> (refnum out=w2365:refnum<file>)  [unwired: 5 in, 2 out]
            n2088 = Open/Create/Replace File "Open File"(file path (use dialog)=w2368) -> (refnum out=w2364:refnum<file>)  [unwired: 5 in, 2 out]
            n2089 = Open/Create/Replace File "Open File"(file path (use dialog)=w2367) -> (refnum out=w2363:refnum<file>)  [unwired: 5 in, 2 out]
            n2090 = while {
              tunnel: w2365 -> [w2387]
              i -> [w2383]
              stop <- w2382 continue-if-true
              (unwired) TRUE ("line mode (F)")
              n2091 = Read from Text File "Read File"(file (use dialog)=w2387) -> (text=w2384:string)  [unwired: 3 in, 3 out]
              n2092 = local write "Numeric 11"(w2383) -> ()
              n2093 = String Length(string=w2384) -> (length=w2386:i32)
              n2094 = Greater?(x=w2386, y=1) -> (0:w2382:bool)
            }
            n2095 = while {
              tunnel: w2364 -> [w2393]
              i -> [w2389]
              stop <- w2388 continue-if-true
              (unwired) TRUE ("line mode (F)")
              n2096 = Read from Text File "Read File"(file (use dialog)=w2393) -> (text=w2390:string)  [unwired: 3 in, 3 out]
              n2097 = local write "Numeric 12"(w2389) -> ()
              n2098 = String Length(string=w2390) -> (length=w2392:i32)
              n2099 = Greater?(x=w2392, y=1) -> (0:w2388:bool)
            }
            n2100 = while {
              tunnel: w2363 -> [w2399]
              i -> [w2395]
              stop <- w2394 continue-if-true
              (unwired) TRUE ("line mode (F)")
              n2101 = Read from Text File "Read File"(file (use dialog)=w2399) -> (text=w2396:string)  [unwired: 3 in, 3 out]
              n2102 = local write "Numeric 13"(w2395) -> ()
              n2103 = String Length(string=w2396) -> (length=w2398:i32)
              n2104 = Greater?(x=w2398, y=1) -> (0:w2394:bool)
            }
            n2105 = String To Path(string=w2362) -> (path=w2370:path)
            n2106 = Open/Create/Replace File "Open File"(file path (use dialog)=w2370) -> (refnum out=w2366:refnum<file>)  [unwired: 5 in, 2 out]
            n2107 = while {
              tunnel: w2366 -> [w2381]
              i -> [w2377]
              stop <- w2376 continue-if-true
              (unwired) TRUE ("line mode (F)")
              n2108 = Read from Text File "Read File"(file (use dialog)=w2381) -> (text=w2378:string)  [unwired: 3 in, 3 out]
              n2109 = local write "Numeric 8"(w2377) -> ()
              n2110 = String Length(string=w2378) -> (length=w2380:i32)
              n2111 = Greater?(x=w2380, y=1) -> (0:w2376:bool)
            }
          }
          frame #1 {
            w2551 = FALSE ("ACTUAL   MERGE")
            # "Sample Temp"
            # "ECR"
            # "COF"
            # "Time\nCOF\nFF\nTemp"
            n2112 = case shown="True" w2424 {
              tunnel: [w2571 w2572] -> w2425
              frame False {
                n2113 = local read "string1"() -> (w2571:string)
              }
              frame True {
                n2114 = local read "String Indicator 4"() -> (w2572:string)
              }
            }
            n2115 = local read "string1 3"() -> (w2469:string)
            n2116 = String To Path(string=w2425) -> (path=w2556:path)
            n2117 = String To Path(string=w2469) -> (path=w2567:path)
            n2118 = local read "Numeric 12"() -> (w2553:i32)
            n2119 = local read "Numeric 8"() -> (w2555:i32)
            n2120 = local read "string1 2"() -> (w2470:string)
            n2121 = local read "string1 4"() -> (w2468:string)
            n2122 = Open/Create/Replace File "Open File"(file path (use dialog)=w2556) -> (refnum out=w2570:refnum<file>, error out=w2569:errorcluster)  [unwired: 5 in, 1 out]
            n2123 = Open/Create/Replace File "Open File"(file path (use dialog)=w2567) -> (refnum out=w2563:refnum<file>, error out=w2564:errorcluster)  [unwired: 5 in, 1 out]
            n2124 = for {
              N: w2555 -> [_]
              tunnel: w2570 -> [w2718]
              tunnel: w2569 -> [w2717]
              tunnel: [w2707] -> w2482 mode=indexing
              tunnel: [w2705] -> w2539 mode=indexing
              tunnel: [w2706] -> w2534 mode=indexing
              tunnel: w2551 -> [_]
              tunnel: [w2699] -> w2536 mode=indexing
              tunnel: [w2695] -> w2505 mode=indexing
              tunnel: [w2691] -> w2480 mode=indexing
              tunnel: [w2687] -> w2461 mode=indexing
              tunnel: [w2682] -> w2421 mode=indexing
              (unwired) TRUE ("line mode (F)")
              # "freq"
              # "Stroke"
              # "Time"
              # "CoF"
              # "Humidity"
              # "Temp"
              # "Air Temp"
              # "ECR"
              n2125 = Read from Text File "Read File"(file (use dialog)=w2718, error in=w2717) -> (text=w2683:string)  [unwired: 2 in, 3 out]
              n2126 = local write "String 6"(w2683) -> ()
              n2127 = String Subset(string=w2683, offset (0)=0, length (rest)=14 ("length (rest)")) -> (substring=w2711:string)
              n2128 = String Subset(string=w2683, offset (0)=35, length (rest)=9 ("length (rest)")) -> (substring=w2708:string)
              n2129 = String Subset(string=w2683, offset (0)=15, length (rest)=9 ("length (rest)")) -> (substring=w2714:string)
              n2130 = Fract/Exp String To Number(string=w2711) -> (number=w2707:dbl)  [unwired: 3 in, 1 out]
              n2131 = Fract/Exp String To Number(string=w2708) -> (number=w2706:dbl)  [unwired: 3 in, 1 out]
              n2132 = Fract/Exp String To Number(string=w2714) -> (number=w2705:dbl)  [unwired: 3 in, 1 out]
              n2133 = String Subset(string=w2683, offset (0)=85, length (rest)=9 ("length (rest)")) -> (substring=w2684:string)
              n2134 = String Subset(string=w2683, offset (0)=25, length (rest)=9 ("length (rest)")) -> (substring=w2690:string)
              n2135 = String Subset(string=w2683, offset (0)=55, length (rest)=9 ("length (rest)")) -> (substring=w2692:string)
              n2136 = String Subset(string=w2683, offset (0)=45, length (rest)=9 ("length (rest)")) -> (substring=w2698:string)
              n2137 = String Subset(string=w2683, offset (0)=65, length (rest)=9 ("length (rest)")) -> (substring=w2704:string)
              n2138 = Fract/Exp String To Number(string=w2690) -> (number=w2687:dbl)  [unwired: 3 in, 1 out]
              n2139 = Fract/Exp String To Number(string=w2684) -> (number=w2682:dbl)  [unwired: 3 in, 1 out]
              n2140 = Fract/Exp String To Number(string=w2692) -> (number=w2691:dbl)  [unwired: 3 in, 1 out]
              n2141 = Fract/Exp String To Number(string=w2698) -> (number=w2695:dbl)  [unwired: 3 in, 1 out]
              n2142 = Fract/Exp String To Number(string=w2704) -> (number=w2701:dbl)  [unwired: 3 in, 1 out]
              n2143 = Add(x=w2701, y=0.0) -> (x+y=w2699:dbl)
            }
            n2144 = for {
              N: w2553 -> [_]
              tunnel: w2564 -> [w2644]
              tunnel: w2563 -> [w2643]
              tunnel: [w2633] -> w2522 mode=indexing
              tunnel: [w2631] -> w2520 mode=indexing
              tunnel: [w2632] -> w2516 mode=indexing
              tunnel: w2551 -> [_]
              tunnel: [w2625] -> w2518 mode=indexing
              tunnel: [w2621] -> w2500 mode=indexing
              tunnel: [w2617] -> w2476 mode=indexing
              tunnel: [w2614] -> w2457 mode=indexing
              tunnel: [w2610] -> w2416 mode=indexing
              (unwired) 9 ("length (rest)")
              (unwired) 9 ("length (rest)")
              (unwired) TRUE ("line mode (F)")
              n2145 = Read from Text File "Read File"(file (use dialog)=w2643, error in=w2644) -> (text=w2611:string)  [unwired: 2 in, 3 out]
              n2146 = local write "String 8"(w2611) -> ()
              n2147 = String Subset(string=w2611, offset (0)=85) -> (substring=w2613:string)  [unwired: 1 in]
              n2148 = String Subset(string=w2611, offset (0)=35, length (rest)=9 ("length (rest)")) -> (substring=w2634:string)
              n2149 = String Subset(string=w2611, offset (0)=55, length (rest)=9 ("length (rest)")) -> (substring=w2619:string)
              n2150 = String Subset(string=w2611, offset (0)=25) -> (substring=w2615:string)  [unwired: 1 in]
              n2151 = String Subset(string=w2611, offset (0)=15, length (rest)=9 ("length (rest)")) -> (substring=w2640:string)
              n2152 = String Subset(string=w2611, offset (0)=0, length (rest)=14 ("length (rest)")) -> (substring=w2637:string)
              n2153 = String Subset(string=w2611, offset (0)=45, length (rest)=9 ("length (rest)")) -> (substring=w2624:string)
              n2154 = String Subset(string=w2611, offset (0)=65, length (rest)=9 ("length (rest)")) -> (substring=w2630:string)
              n2155 = Fract/Exp String To Number(string=w2613) -> (number=w2610:dbl)  [unwired: 3 in, 1 out]
              n2156 = Fract/Exp String To Number(string=w2634) -> (number=w2632:dbl)  [unwired: 3 in, 1 out]
              n2157 = Fract/Exp String To Number(string=w2619) -> (number=w2617:dbl)  [unwired: 3 in, 1 out]
              n2158 = Fract/Exp String To Number(string=w2615) -> (number=w2614:dbl)  [unwired: 3 in, 1 out]
              n2159 = Fract/Exp String To Number(string=w2640) -> (number=w2631:dbl)  [unwired: 3 in, 1 out]
              n2160 = Fract/Exp String To Number(string=w2637) -> (number=w2633:dbl)  [unwired: 3 in, 1 out]
              n2161 = Fract/Exp String To Number(string=w2624) -> (number=w2621:dbl)  [unwired: 3 in, 1 out]
              n2162 = Fract/Exp String To Number(string=w2630) -> (number=w2627:dbl)  [unwired: 3 in, 1 out]
              n2163 = Add(x=w2627, y=0.0) -> (x+y=w2625:dbl)
            }
            n2164 = String To Path(string=w2470) -> (path=w2568:path)
            n2165 = String To Path(string=w2468) -> (path=w2562:path)
            n2166 = local read "Numeric 11"() -> (w2552:i32)
            n2167 = local read "Numeric 13"() -> (w2554:i32)
            n2168 = Open/Create/Replace File "Open File"(file path (use dialog)=w2568) -> (refnum out=w2566:refnum<file>, error out=w2565:errorcluster)  [unwired: 5 in, 1 out]
            n2169 = Open/Create/Replace File "Open File"(file path (use dialog)=w2562) -> (refnum out=w2561:refnum<file>, error out=w2560:errorcluster)  [unwired: 5 in, 1 out]
            n2170 = for {
              N: w2552 -> [_]
              tunnel: w2566 -> [w2681]
              tunnel: w2565 -> [w2680]
              tunnel: [w2670] -> w2532 mode=indexing
              tunnel: [w2668] -> w2530 mode=indexing
              tunnel: [w2669] -> w2525 mode=indexing
              tunnel: w2551 -> [_]
              tunnel: [w2662] -> w2527 mode=indexing
              tunnel: [w2658] -> w2503 mode=indexing
              tunnel: [w2654] -> w2478 mode=indexing
              tunnel: [w2650] -> w2459 mode=indexing
              tunnel: [w2645] -> w2417 mode=indexing
              (unwired) TRUE ("line mode (F)")
              n2171 = Read from Text File "Read File"(file (use dialog)=w2681, error in=w2680) -> (text=w2646:string)  [unwired: 2 in, 3 out]
              n2172 = local write "String 7"(w2646) -> ()
              n2173 = String Subset(string=w2646, offset (0)=85, length (rest)=9 ("length (rest)")) -> (substring=w2649:string)
              n2174 = String Subset(string=w2646, offset (0)=35, length (rest)=9 ("length (rest)")) -> (substring=w2671:string)
              n2175 = String Subset(string=w2646, offset (0)=55, length (rest)=9 ("length (rest)")) -> (substring=w2657:string)
              n2176 = String Subset(string=w2646, offset (0)=25, length (rest)=9 ("length (rest)")) -> (substring=w2651:string)
              n2177 = String Subset(string=w2646, offset (0)=45, length (rest)=9 ("length (rest)")) -> (substring=w2659:string)
              n2178 = String Subset(string=w2646, offset (0)=0, length (rest)=14 ("length (rest)")) -> (substring=w2674:string)
              n2179 = String Subset(string=w2646, offset (0)=15, length (rest)=9 ("length (rest)")) -> (substring=w2677:string)
              n2180 = String Subset(string=w2646, offset (0)=65, length (rest)=9 ("length (rest)")) -> (substring=w2663:string)
              n2181 = Fract/Exp String To Number(string=w2649) -> (number=w2645:dbl)  [unwired: 3 in, 1 out]
              n2182 = Fract/Exp String To Number(string=w2671) -> (number=w2669:dbl)  [unwired: 3 in, 1 out]
              n2183 = Fract/Exp String To Number(string=w2657) -> (number=w2654:dbl)  [unwired: 3 in, 1 out]
              n2184 = Fract/Exp String To Number(string=w2651) -> (number=w2650:dbl)  [unwired: 3 in, 1 out]
              n2185 = Fract/Exp String To Number(string=w2659) -> (number=w2658:dbl)  [unwired: 3 in, 1 out]
              n2186 = Fract/Exp String To Number(string=w2674) -> (number=w2670:dbl)  [unwired: 3 in, 1 out]
              n2187 = Fract/Exp String To Number(string=w2677) -> (number=w2668:dbl)  [unwired: 3 in, 1 out]
              n2188 = Fract/Exp String To Number(string=w2663) -> (number=w2666:dbl)  [unwired: 3 in, 1 out]
              n2189 = Add(x=w2666, y=0.0) -> (x+y=w2662:dbl)
            }
            n2190 = for {
              N: w2554 -> [_]
              tunnel: w2561 -> [w2609]
              tunnel: w2560 -> [w2608]
              tunnel: [w2598] -> w2514 mode=indexing
              tunnel: [w2597] -> w2507 mode=indexing
              tunnel: w2551 -> [_]
              tunnel: [w2586] -> w2512 mode=indexing
              tunnel: [w2591] -> w2509 mode=indexing
              tunnel: [w2587] -> w2499 mode=indexing
              tunnel: [w2582] -> w2474 mode=indexing
              tunnel: [w2578] -> w2455 mode=indexing
              tunnel: [w2573] -> w2415 mode=indexing
              (unwired) 1.0 ("x")
              (unwired) TRUE ("line mode (F)")
              n2191 = Read from Text File "Read File"(file (use dialog)=w2609, error in=w2608) -> (text=w2574:string)  [unwired: 2 in, 3 out]
              n2192 = local write "String 12"(w2574) -> ()
              n2193 = String Subset(string=w2574, offset (0)=85, length (rest)=9 ("length (rest)")) -> (substring=w2576:string)
              n2194 = String Subset(string=w2574, offset (0)=35, length (rest)=9 ("length (rest)")) -> (substring=w2599:string)
              n2195 = String Subset(string=w2574, offset (0)=55, length (rest)=9 ("length (rest)")) -> (substring=w2584:string)
              n2196 = String Subset(string=w2574, offset (0)=25, length (rest)=9 ("length (rest)")) -> (substring=w2580:string)
              n2197 = String Subset(string=w2574, offset (0)=45, length (rest)=9 ("length (rest)")) -> (substring=w2589:string)
              n2198 = String Subset(string=w2574, offset (0)=15, length (rest)=9 ("length (rest)")) -> (substring=w2605:string)
              n2199 = String Subset(string=w2574, offset (0)=0, length (rest)=14 ("length (rest)")) -> (substring=w2602:string)
              n2200 = String Subset(string=w2574, offset (0)=65, length (rest)=9 ("length (rest)")) -> (substring=w2592:string)
              n2201 = Fract/Exp String To Number(string=w2576) -> (number=w2573:dbl)  [unwired: 3 in, 1 out]
              n2202 = Fract/Exp String To Number(string=w2599) -> (number=w2597:dbl)  [unwired: 3 in, 1 out]
              n2203 = Fract/Exp String To Number(string=w2584) -> (number=w2582:dbl)  [unwired: 3 in, 1 out]
              n2204 = Fract/Exp String To Number(string=w2580) -> (number=w2578:dbl)  [unwired: 3 in, 1 out]
              n2205 = Fract/Exp String To Number(string=w2589) -> (number=w2587:dbl)  [unwired: 3 in, 1 out]
              n2206 = Fract/Exp String To Number(string=w2605) -> (number=w2586:dbl)  [unwired: 3 in, 1 out]
              n2207 = Fract/Exp String To Number(string=w2602) -> (number=w2598:dbl)  [unwired: 3 in, 1 out]
              n2208 = Fract/Exp String To Number(string=w2592) -> (number=w2595:dbl)  [unwired: 3 in, 1 out]
              n2209 = Add(x=w2595, y=0.0) -> (x+y=w2591:dbl)
            }
            n2210 = Delete From Array(array=w2457, index=0) -> (array with subset deleted=w2430:dbl[])  [unwired: 1 in, 1 out]
            n2211 = Delete From Array(array=w2520, index=0) -> (array with subset deleted=w2493:dbl[])  [unwired: 1 in, 1 out]
            n2212 = Delete From Array(array=w2500, index=0) -> (array with subset deleted=w2488:dbl[])  [unwired: 1 in, 1 out]
            n2213 = Delete From Array(array=w2518, index=0) -> (array with subset deleted=w2519:dbl[])  [unwired: 1 in, 1 out]
            n2214 = call-poly <vilib>:"Mean.vi"("X"=w2430) -> ("mean"=→"КОФ2 4":dbl)  [unwired: 1 out]
            n2215 = call-poly <vilib>:"Mean.vi"("X"=w2493) -> ("mean"=→"КОФ3":dbl)  [unwired: 1 out]
            n2216 = call-poly <vilib>:"Mean.vi"("X"=w2488) -> ("mean"=→"CP3":dbl)  [unwired: 1 out]
            n2217 = Delete From Array(array=w2482, index=0) -> (array with subset deleted=w2409:dbl[])  [unwired: 1 in, 1 out]